vi "Dresden R2R Sputter 03.02.2018 IY24.vi"() -> ()   [LabVIEW 2009] (continued)
                                frame #0 {
                                n25284 = local read "R Set Pressure mtorr"() -> (w30584:dbl)
                                n25285 = local write "Set_pressure_value 2"(w30584) -> ()
                                }
                                frame #1 {
                                }
                                }
                                }
                                frame #1 {
                                n25286 = local read "Semi"() -> (w30585:bool)
                                n25287 = case shown="False" w30585 {
                                frame #0 {
                                n25288 = Wait (ms)(milliseconds to wait=u32 1000) -> ()  [unwired: 1 out]
                                }
                                frame #1 {
                                }
                                }
                                }
                                frame #2 {
                                n25289 = local read "Semi"() -> (w30587:bool)
                                n25290 = case shown="False" w30587 {
                                frame #0 {
                                n25291 = local write "Pc_bv2_auto_set_pressure"(TRUE ("Pc_bv1_auto_set_pressure")) -> ()
                                }
                                frame #1 {
                                }
                                }
                                }
                                frame #3 {
                                n25292 = local read "Semi"() -> (w30589:bool)
                                n25293 = case shown="False" w30589 {
                                frame #0 {
                                n25294 = while {
                                i -> [w30600]
                                stop <- w30592 stop-if-true
                                n25295 = Greater?(x=w30600, y=300) -> (0:w30594:bool)
                                n25296 = local read "Set_pressure_value 2"() -> (w30590:dbl)
                                n25297 = Add(x=1.0, y=w30590) -> (x+y=w30596:dbl)
                                n25298 = Subtract(x=w30590, y=1.0) -> (x-y=w30597:dbl)
                                n25299 = local read "Pressure 2"() -> (w30591:i32)
                                n25300 = In Range and Coerce(upper limit=w30596, x=w30591, lower limit=w30597) -> (In Range?=w30595:bool)  [unwired: 1 out]
                                n25301 = case shown="False" w30595 {
                                tunnel: [FALSE TRUE] -> w30593
                                frame #0 {
                                n25302 = Wait Until Next ms Multiple(millisecond multiple=u32 200) -> ()  [unwired: 1 out]
                                }
                                frame #1 {
                                }
                                }
                                n25303 = Or(x=w30593, y=w30594) -> (x .or. y?=w30592:bool)
                                }
                                }
                                frame #1 {
                                }
                                }
                                }
                                frame #4 {
                                n25304 = local read "Semi"() -> (w30605:bool)
                                n25305 = case shown="False" w30605 {
                                frame #0 {
                                n25306 = local read "Set_pressure_value 2"() -> (w30606:dbl)
                                n25307 = Add(x=1.0, y=w30606) -> (x+y=w30609:dbl)
                                n25308 = Subtract(x=w30606, y=1.0) -> (x-y=w30610:dbl)
                                n25309 = local read "Pressure 2"() -> (w30607:i32)
                                n25310 = In Range and Coerce(upper limit=w30609, x=w30607, lower limit=w30610) -> (In Range?=w30608:bool)  [unwired: 1 out]
                                n25311 = case shown="False" w30608 {
                                frame #0 {
                                n25312 = local read "R Set Pressure mtorr"() -> (w30613:dbl)
                                n25313 = local write "Set_pressure_value 2"(w30613) -> ()
                                }
                                frame #1 {
                                }
                                }
                                }
                                frame #1 {
                                }
                                }
                                }
                                frame #5 {
                                n25314 = local read "Semi"() -> (w30614:bool)
                                n25315 = case shown="False" w30614 {
                                frame #0 {
                                n25316 = local read "Set_pressure_value 2"() -> (w30615:dbl)
                                n25317 = Add(x=1.0, y=w30615) -> (x+y=w30618:dbl)
                                n25318 = Subtract(x=w30615, y=1.0) -> (x-y=w30619:dbl)
                                n25319 = local read "Pressure 2"() -> (w30616:i32)
                                n25320 = In Range and Coerce(upper limit=w30618, x=w30616, lower limit=w30619) -> (In Range?=w30617:bool)  [unwired: 1 out]
                                n25321 = case shown="False" w30617 {
                                frame #0 {
                                n25322 = local write "Pc_bv2_auto_set_pressure"(TRUE ("Pc_bv1_auto_set_pressure")) -> ()
                                }
                                frame #1 {
                                }
                                }
                                }
                                frame #1 {
                                }
                                }
                                }
                                frame #6 {
                                n25323 = local read "Semi"() -> (w30623:bool)
                                n25324 = case shown="False" w30623 {
                                frame #0 {
                                n25325 = while {
                                i -> [w30634]
                                stop <- w30625 stop-if-true
                                n25326 = Greater?(x=w30634, y=300) -> (0:w30627:bool)
                                n25327 = local read "Set_pressure_value 2"() -> (w30629:dbl)
                                n25328 = Add(x=1.0, y=w30629) -> (x+y=w30630:dbl)
                                n25329 = Subtract(x=w30629, y=1.0) -> (x-y=w30631:dbl)
                                n25330 = local read "Pressure 2"() -> (w30624:i32)
                                n25331 = In Range and Coerce(upper limit=w30630, x=w30624, lower limit=w30631) -> (In Range?=w30628:bool)  [unwired: 1 out]
                                n25332 = case shown="False" w30628 {
                                tunnel: [FALSE TRUE] -> w30626
                                frame #0 {
                                n25333 = Wait Until Next ms Multiple(millisecond multiple=u32 200) -> ()  [unwired: 1 out]
                                }
                                frame #1 {
                                }
                                }
                                n25334 = Or(x=w30626, y=w30627) -> (x .or. y?=w30625:bool)
                                }
                                }
                                frame #1 {
                                }
                                }
                                }
                                frame #7 {
                                n25335 = local read "Semi"() -> (w30639:bool)
                                n25336 = case shown="False" w30639 {
                                frame #0 {
                                n25337 = local read "Set_pressure_value 2"() -> (w30642:dbl)
                                n25338 = Add(x=1.0, y=w30642) -> (x+y=w30643:dbl)
                                n25339 = Subtract(x=w30642, y=1.0) -> (x-y=w30644:dbl)
                                n25340 = local read "Pressure 2"() -> (w30640:i32)
                                n25341 = In Range and Coerce(upper limit=w30643, x=w30640, lower limit=w30644) -> (In Range?=w30641:bool)  [unwired: 1 out]
                                n25342 = case shown="False" w30641 {
                                frame #0 {
                                n25343 = local write "Semi"(TRUE ("Semi")) -> ()
                                n25344 = local write "Error Message"("Coating Pressure could not be adjusted !" ("Error Message")) -> ()
                                }
                                frame #1 {
                                }
                                }
                                }
                                frame #1 {
                                }
                                }
                                }
                                }
                                }
                                frame #1 {
                                }
                                }
                                }
                                frame #1 {
                                n25345 = local read "Semi"() -> (w30649:bool)
                                n25346 = case shown="False" w30649 {
                                frame #0 {
                                n25347 = local write "SDC1 9"(TRUE ("SDC1 9")) -> ()
                                n25348 = Wait (ms)(milliseconds to wait=u32 1000) -> ()  [unwired: 1 out]
                                }
                                frame #1 {
                                }
                                }
                                }
                                }
                                }
                                }
                                }
                                frame #15 {
                                # "DC -Ignite Plasma"
                                n25349 = stacked-sequence {
                                frame #0 {
                                n25350 = local read "Semi"() -> (w30652:bool)
                                n25351 = case shown="False" w30652 {
                                frame #0 {
                                n25352 = stacked-sequence {
                                frame #0 {
                                n25353 = local read "Semi"() -> (w30653:bool)
                                n25354 = case shown="False" w30653 {
                                frame #0 {
                                n25355 = while {
                                i -> [w30659]
                                stop <- w30654 stop-if-true
                                n25356 = Greater?(x=w30659, y=50) -> (0:w30658:bool)
                                n25357 = case shown="True" w30658 {
                                frame #0 {
                                }
                                frame #1 {
                                n25358 = local write "Semi"(TRUE ("Semi")) -> ()
                                n25359 = local write "Error Message"("Sputtering Process cancelled.\nPlease check \nDC switch connections." ("Error Message")) -> ()
                                }
                                }
                                n25360 = local read "Cnt_Dcps_sw2_di"() -> (w30657:bool)
                                n25361 = case shown="True" w30657 {
                                tunnel: [TRUE ("Cnt_Dcps_sw1_do") FALSE ("Cnt_Dcps_sw1_do")] -> w30656
                                frame #0 {
                                }
                                frame #1 {
                                n25362 = local write "Cnt_Dcps_sw2_do"(FALSE ("Cnt_Dcps_sw1_do")) -> ()
                                n25363 = Wait Until Next ms Multiple(millisecond multiple=u32 200) -> ()  [unwired: 1 out]
                                }
                                }
                                n25364 = local read "Semi"() -> (w30655:bool)
                                n25365 = Or(x=w30656, y=w30655) -> (x .or. y?=w30654:bool)
                                }
                                }
                                frame #1 {
                                }
                                }
                                }
                                frame #1 {
                                n25366 = local read "Semi"() -> (w30667:bool)
                                n25367 = case shown="False" w30667 {
                                frame #0 {
                                n25368 = while {
                                i -> [w30673]
                                stop <- w30668 stop-if-true
                                n25369 = Greater?(x=w30673, y=50) -> (0:w30672:bool)
                                n25370 = case shown="True" w30672 {
                                frame #0 {
                                }
                                frame #1 {
                                n25371 = local write "Semi"(TRUE ("Semi")) -> ()
                                n25372 = local write "Error Message"("Sputtering Process cancelled.\nPlease check \nDC switch connections." ("Error Message")) -> ()
                                }
                                }
                                n25373 = local read "Cnt_Dcps_sw1_di"() -> (w30671:bool)
                                n25374 = case shown="False" w30671 {
                                tunnel: [FALSE ("Cnt_Dcps_sw1_do") TRUE ("Cnt_Dcps_sw1_do")] -> w30670
                                frame #0 {
                                n25375 = local write "Cnt_Dcps_sw1_do"(TRUE ("Cnt_Dcps_sw1_do")) -> ()
                                n25376 = Wait Until Next ms Multiple(millisecond multiple=u32 200) -> ()  [unwired: 1 out]
                                }
                                frame #1 {
                                }
                                }
                                n25377 = local read "Semi"() -> (w30669:bool)
                                n25378 = Or(x=w30670, y=w30669) -> (x .or. y?=w30668:bool)
                                }
                                }
                                frame #1 {
                                }
                                }
                                }
                                frame #2 {
                                n25379 = local read "Semi"() -> (w30681:bool)
                                n25380 = case shown="False" w30681 {
                                frame #0 {
                                n25381 = local write "Dc_host_auto"(TRUE ("Dc_host_auto")) -> ()
                                }
                                frame #1 {
                                }
                                }
                                }
                                frame #3 {
                                n25382 = local read "Semi"() -> (w30683:bool)
                                n25383 = case shown="False" w30683 {
                                frame #0 {
                                n25384 = local read "R Single DC Step1 Coating Power"() -> (w30684:dbl)
                                n25385 = local write "Set DC Power       :"(w30684) -> ()
                                }
                                frame #1 {
                                }
                                }
                                }
                                frame #4 {
                                n25386 = local read "Semi"() -> (w30685:bool)
                                n25387 = case shown="False" w30685 {
                                frame #0 {
                                n25388 = Wait (ms)(milliseconds to wait=u32 1000) -> ()  [unwired: 1 out]
                                }
                                frame #1 {
                                }
                                }
                                }
                                frame #5 {
                                n25389 = local read "Semi"() -> (w30687:bool)
                                n25390 = case shown="False" w30687 {
                                frame #0 {
                                n25391 = local write "Dc_auto_set"(TRUE ("Dc_auto_set")) -> ()
                                }
                                frame #1 {
                                }
                                }
                                }
                                frame #6 {
                                n25392 = Wait (ms)(milliseconds to wait=u32 1000) -> ()  [unwired: 1 out]
                                }
                                frame #7 {
                                n25393 = local read "Semi"() -> (w30690:bool)
                                n25394 = case shown="False" w30690 {
                                frame #0 {
                                n25395 = local read "Web_selection_tab"() -> (w30691:T5)
                                n25396 = case shown="\"Other                                                                                    \"" w30691 {
                                frame #0 {
                                }
                                frame #1 {
                                n25397 = local write "Dc_auto_on"(TRUE ("Dc_auto_on")) -> ()
                                }
                                }
                                }
                                frame #1 {
                                }
                                }
                                }
                                frame #8 {
                                n25398 = local read "Web_selection_tab"() -> (w30693:T5)
                                n25399 = case shown="\"Other                                                                                    \"" w30693 {
                                frame #0 {
                                }
                                frame #1 {
                                n25400 = local read "Semi"() -> (w30694:bool)
                                n25401 = case shown="False" w30694 {
                                frame #0 {
                                n25402 = while {
                                i -> [w30704]
                                stop <- w30695 stop-if-true
                                n25403 = Greater Or Equal?(x=w30704, y=240) -> (x >= y?=w30703:bool)
                                n25404 = case shown="True" w30703 {
                                frame #0 {
                                }
                                frame #1 {
                                n25405 = local write "Semi"(TRUE ("Semi")) -> ()
                                }
                                }
                                n25406 = local read "Set DC Power       :"() -> (w30700:dbl)
                                n25407 = local read "Actual DC Power"() -> (w30699:dbl)
                                n25408 = Subtract(x=w30700, y=w30699) -> (x-y=w30702:dbl)
                                n25409 = Less?(x=w30702, y=10.0) -> (x < y?=w30697:bool)
                                n25410 = local read "Semi"() -> (w30696:bool)
                                n25411 = Or(x=w30697, y=w30696) -> (x .or. y?=w30695:bool)
                                n25412 = Wait Until Next ms Multiple(millisecond multiple=u32 500) -> ()  [unwired: 1 out]
                                }
                                }
                                frame #1 {
                                }
                                }
                                }
                                }
                                }
                                frame #9 {
                                n25413 = local read "Semi"() -> (w30707:bool)
                                n25414 = case shown="False" w30707 {
                                frame #0 {
                                n25415 = Wait (ms)(milliseconds to wait=u32 1000) -> ()  [unwired: 1 out]
                                }
                                frame #1 {
                                }
                                }
                                }
                                }
                                }
                                frame #1 {
                                }
                                }
                                }
                                frame #1 {
                                n25416 = local read "Semi"() -> (w30709:bool)
                                n25417 = case shown="False" w30709 {
                                frame #0 {
                                n25418 = Wait (ms)(milliseconds to wait=u32 1000) -> ()  [unwired: 1 out]
                                n25419 = local write "SDC1 13"(TRUE ("SDC1 13")) -> ()
                                }
                                frame #1 {
                                }
                                }
                                }
                                }
                                }
                                frame #16 {
                                n25420 = local read "Web_selection_tab"() -> (w30712:T5)
                                n25421 = case shown="\"Web                                                                                    \", Default" w30712 {
                                frame #0 {
                                n25422 = stacked-sequence {
                                frame #0 {
                                n25423 = local read "R Web speed(cm/min)"() -> (w30716:dbl)
                                n25424 = local read "R Minimum diameter"() -> (w30713:dbl)
                                n25425 = local read "R Maximum diameter"() -> (w30714:dbl)
                                n25426 = local read "R Web thicness"() -> (w30715:dbl)
                                n25427 = local write "Initial Min Diameter"(w30713) -> ()
                                n25428 = local write "Web Thickness"(w30715) -> ()
                                n25429 = local write "Max Diameter"(w30714) -> ()
                                n25430 = local write "Web Speed"(w30716) -> ()
                                n25431 = Wait (ms)(milliseconds to wait=u32 100) -> ()  [unwired: 1 out]
                                }
                                frame #1 {
                                n25432 = local read "R Single DC Step1 Coating Power Active"() -> (w30731:bool)
                                n25433 = local read "R Single DC Step2 Coating Power Active"() -> (w30730:bool)
                                n25434 = local read "R Single DC Step3 Coating Power Active"() -> (w30729:bool)
                                n25435 = local read "R Single DC Step4 Coating Power Active"() -> (w30728:bool)
                                n25436 = local read "R Single DC Step5 Coating Power Active"() -> (w30727:bool)
                                n25437 = Boolean To (0,1)(Boolean=w30731) -> (0, 1=w30726:i16)
                                n25438 = Boolean To (0,1)(Boolean=w30730) -> (0, 1=w30725:i16)
                                n25439 = Boolean To (0,1)(Boolean=w30729) -> (0, 1=w30724:i16)
                                n25440 = Boolean To (0,1)(Boolean=w30728) -> (0, 1=w30723:i16)
                                n25441 = Boolean To (0,1)(Boolean=w30727) -> (0, 1=w30722:i16)
                                n25442 = Compound Arithmetic op=ADD(w30726, w30725, w30724, w30723, w30722) -> (w30720:i16)
                                n25443 = local read "R Single DC Interval length"() -> (w30721:dbl)
                                n25444 = Wait (ms)(milliseconds to wait=u32 200) -> ()  [unwired: 1 out]
                                n25445 = Multiply(x=w30721, y=w30720) -> (x*y=w30719:dbl)
                                n25446 = local write "Total length"(w30719) -> ()
                                }
                                frame #2 {
                                n25447 = local write "Calculate 2"(TRUE ("Calculate_auto")) -> ()
                                }
                                frame #3 {
                                n25448 = local write "Roll_side_select"(enum32{"Left to Right", "Right to Left"}."Left to Right" ("Roll_side_select")) -> ()
                                }
                                frame #4 {
                                n25449 = Wait (ms)(milliseconds to wait=u32 100) -> ()  [unwired: 1 out]
                                n25450 = local write "Parameters_auto_set"(TRUE ("Parameters_auto_set")) -> ()
                                }
                                frame #5 {
                                n25451 = while {
                                i -> [w30740]
                                stop <- w30736 stop-if-true
                                n25452 = Wait Until Next ms Multiple(millisecond multiple=u32 300) -> ()  [unwired: 1 out]
                                n25453 = Greater?(x=w30740, y=100) -> (0:w30737:bool)
                                n25454 = local read "Parameters_auto_set"() -> (w30741:bool)
                                n25455 = case shown="False" w30741 {
                                tunnel: [TRUE FALSE] -> w30738
                                frame #0 {
                                }
                                frame #1 {
                                }
                                }
                                n25456 = Or(x=w30738, y=w30737) -> (x .or. y?=w30736:bool)
                                }
                                }
                                frame #6 {
                                n25457 = local read "R Tension Value"() -> (w30745:dbl)
                                n25458 = Wait (ms)(milliseconds to wait=u32 200) -> ()  [unwired: 1 out]
                                n25459 = local write "TC1_set_value"(w30745) -> ()
                                }
                                frame #7 {
                                n25460 = local write "TC1_auto_set"(TRUE ("TC1_auto_set")) -> ()
                                }
                                frame #8 {
                                w30749 = u16 1 items=["1", "2", "3", "4"] ("Target Chamber Sensor")
                                n25461 = local write "Target Chamber Sensor"(w30749) -> ()
                                n25462 = Wait (ms)(milliseconds to wait=u32 200) -> ()  [unwired: 1 out]
                                }
                                frame #9 {
                                n25463 = local read "Total length"() -> (w30750:dbl)
                                n25464 = local write "Region"(w30750) -> ()
                                }
                                frame #10 {
                                n25465 = local read "Semi"() -> (w30751:bool)
                                n25466 = case shown="False" w30751 {
                                frame #0 {
                                n25467 = stacked-sequence {
                                frame #0 {
                                # "Gas Flow"
                                n25468 = stacked-sequence {
                                frame #0 {
                                n25469 = local read "Semi"() -> (w30752:bool)
                                n25470 = case shown="False" w30752 {
                                frame #0 {
                                n25471 = stacked-sequence {
                                frame #0 {
                                n25472 = local read "Semi"() -> (w30753:bool)
                                n25473 = case shown="False" w30753 {
                                frame #0 {
                                n25474 = local read "R Argon Flow sccm"() -> (w30754:dbl)
                                n25475 = local write "Ar_sccm1_2"(w30754) -> ()
                                }
                                frame #1 {
                                }
                                }
                                }
                                frame #1 {
                                n25476 = local read "Semi"() -> (w30755:bool)
                                n25477 = case shown="False" w30755 {
                                frame #0 {
                                n25478 = local write "Mfc_Ar _1_2_set"(TRUE ("Mfc_Ar _1_2_set")) -> ()
                                }
                                frame #1 {
                                }
                                }
                                }
                                frame #2 {
                                n25479 = local read "Semi"() -> (w30757:bool)
                                n25480 = case shown="False" w30757 {
                                frame #0 {
                                n25481 = while {
                                i -> [w30760]
                                stop <- w30762 stop-if-true
                                n25482 = Greater?(x=w30760, y=50) -> (0:w30759:bool)
                                n25483 = local read "Semi"() -> (w30758:bool)
                                n25484 = Or(x=w30758, y=w30759) -> (x .or. y?=w30762:bool)
                                }
                                }
                                frame #1 {
                                }
                                }
                                }
                                frame #3 {
                                n25485 = local read "Semi"() -> (w30763:bool)
                                n25486 = case shown="False" w30763 {
                                frame #0 {
                                n25487 = local read "Ar_sccm_act 6"() -> (w30764:dbl)
                                n25488 = Greater?(x=w30764, y=1) -> (0:w30765:bool)
                                n25489 = case shown="False" w30765 {
                                frame #0 {
                                n25490 = local read "R Argon Flow sccm"() -> (w30767:dbl)
                                n25491 = local write "Ar_sccm1_2"(w30767) -> ()
                                }
                                frame #1 {
                                }
                                }
                                }
                                frame #1 {
                                }
                                }
                                }
                                frame #4 {
                                n25492 = local read "Semi"() -> (w30768:bool)
                                n25493 = case shown="False" w30768 {
                                frame #0 {
                                n25494 = local read "Ar_sccm_act 6"() -> (w30770:dbl)
                                n25495 = Greater?(x=w30770, y=1) -> (0:w30769:bool)
                                n25496 = case shown="False" w30769 {
                                frame #0 {
                                n25497 = while {
                                i -> [w30773]
                                stop <- w30777 stop-if-true
                                n25498 = Greater?(x=w30773, y=50) -> (0:w30772:bool)
                                n25499 = local read "Semi"() -> (w30776:bool)
                                n25500 = case shown="False" w30776 {
                                tunnel: [FALSE TRUE] -> w30775
                                frame #0 {
                                n25501 = Wait Until Next ms Multiple(millisecond multiple=u32 200) -> ()  [unwired: 1 out]
                                }
                                frame #1 {
                                }
                                }
                                n25502 = Or(x=w30775, y=w30772) -> (x .or. y?=w30777:bool)
                                }
                                }
                                frame #1 {
                                }
                                }
                                }
                                frame #1 {
                                }
                                }
                                }
                                frame #5 {
                                n25503 = local read "Semi"() -> (w30781:bool)
                                n25504 = case shown="False" w30781 {
                                frame #0 {
                                n25505 = local read "Ar_sccm_act 5"() -> (w30783:dbl)
                                n25506 = Greater?(x=w30783, y=1) -> (0:w30782:bool)
                                n25507 = case shown="False" w30782 {
                                frame #0 {
                                n25508 = local write "Semi"(TRUE ("Semi")) -> ()
                                n25509 = local write "Error Message"("Coating process cancelled.\nPlease check connections." ("Error Message")) -> ()
                                }
                                frame #1 {
                                }
                                }
                                }
                                frame #1 {
                                }
                                }
                                }
                                }
                                }
                                frame #1 {
                                }
                                }
                                }
                                frame #1 {
                                n25510 = local read "Semi"() -> (w30787:bool)
                                n25511 = case shown="False" w30787 {
                                frame #0 {
                                n25512 = local write "SDC1 11"(TRUE ("SDC1 11")) -> ()
                                n25513 = Wait (ms)(milliseconds to wait=u32 1000) -> ()  [unwired: 1 out]
                                }
                                frame #1 {
                                }
                                }
                                }
                                }
                                }
                                frame #1 {
                                # "Set Pressure for ignite plasma"
                                n25514 = stacked-sequence {
                                frame #0 {
                                n25515 = local read "Semi"() -> (w30790:bool)
                                n25516 = case shown="False" w30790 {
                                frame #0 {
                                n25517 = stacked-sequence {
                                frame #0 {
                                n25518 = local read "Semi"() -> (w30791:bool)
                                n25519 = case shown="False" w30791 {
                                frame #0 {
                                n25520 = local write "Set_pressure_value 2"(10.0 ("Set_pressure_value 2")) -> ()
                                }
                                frame #1 {
                                }
                                }
                                }
                                frame #1 {
                                n25521 = local read "Semi"() -> (w30793:bool)
                                n25522 = case shown="False" w30793 {
                                frame #0 {
                                n25523 = Wait (ms)(milliseconds to wait=u32 1000) -> ()  [unwired: 1 out]
                                }
                                frame #1 {
                                }
                                }
                                }
                                frame #2 {
                                n25524 = local read "Semi"() -> (w30795:bool)
                                n25525 = case shown="False" w30795 {
                                frame #0 {
                                n25526 = local write "Pc_bv2_auto_set_pressure"(TRUE ("Pc_bv1_auto_set_pressure")) -> ()
                                }
                                frame #1 {
                                }
                                }
                                }
                                frame #3 {
                                n25527 = local read "Semi"() -> (w30797:bool)
                                n25528 = case shown="False" w30797 {
                                frame #0 {
                                n25529 = while {
                                i -> [w30808]
                                stop <- w30800 stop-if-true
                                w30798 = 10.0 ("Set_pressure_value 2")
                                n25530 = Greater?(x=w30808, y=300) -> (0:w30802:bool)
                                n25531 = Add(x=1.0, y=w30798) -> (x+y=w30804:dbl)
                                n25532 = Subtract(x=w30798, y=1.0) -> (x-y=w30805:dbl)
                                n25533 = local read "Pressure 2"() -> (w30799:i32)
                                n25534 = In Range and Coerce(upper limit=w30804, x=w30799, lower limit=w30805) -> (In Range?=w30803:bool)  [unwired: 1 out]
                                n25535 = case shown="False" w30803 {
                                tunnel: [FALSE TRUE] -> w30801
                                frame #0 {
                                n25536 = Wait Until Next ms Multiple(millisecond multiple=u32 200) -> ()  [unwired: 1 out]
                                }
                                frame #1 {
                                }
                                }
                                n25537 = Or(x=w30801, y=w30802) -> (x .or. y?=w30800:bool)
                                }
                                }
                                frame #1 {
                                }
                                }
                                }
                                frame #4 {
                                n25538 = local read "Semi"() -> (w30813:bool)
                                n25539 = case shown="False" w30813 {
                                frame #0 {
                                w30814 = 10.0 ("Set_pressure_value 2")
                                n25540 = Add(x=1.0, y=w30814) -> (x+y=w30817:dbl)
                                n25541 = Subtract(x=w30814, y=1.0) -> (x-y=w30818:dbl)
                                n25542 = local read "Pressure 2"() -> (w30815:i32)
                                n25543 = In Range and Coerce(upper limit=w30817, x=w30815, lower limit=w30818) -> (In Range?=w30816:bool)  [unwired: 1 out]
                                n25544 = case shown="False" w30816 {
                                frame #0 {
                                n25545 = local read "R Set Pressure mtorr"() -> (w30821:dbl)
                                n25546 = local write "Set_pressure_value 2"(w30821) -> ()
                                }
                                frame #1 {
                                }
                                }
                                }
                                frame #1 {
                                }
                                }
                                }
                                frame #5 {
                                n25547 = local read "Semi"() -> (w30822:bool)
                                n25548 = case shown="False" w30822 {
                                frame #0 {
                                w30823 = 10.0 ("Set_pressure_value 2")
                                n25549 = Add(x=1.0, y=w30823) -> (x+y=w30826:dbl)
                                n25550 = Subtract(x=w30823, y=1.0) -> (x-y=w30827:dbl)
                                n25551 = local read "Pressure 2"() -> (w30824:i32)
                                n25552 = In Range and Coerce(upper limit=w30826, x=w30824, lower limit=w30827) -> (In Range?=w30825:bool)  [unwired: 1 out]
                                n25553 = case shown="False" w30825 {
                                frame #0 {
                                n25554 = local write "Pc_bv2_auto_set_pressure"(TRUE ("Pc_bv1_auto_set_pressure")) -> ()
                                }
                                frame #1 {
                                }
                                }
                                }
                                frame #1 {
                                }
                                }
                                }
                                frame #6 {
                                n25555 = local read "Semi"() -> (w30831:bool)
                                n25556 = case shown="False" w30831 {
                                frame #0 {
                                n25557 = while {
                                i -> [w30842]
                                stop <- w30834 stop-if-true
                                w30832 = 10.0 ("Set_pressure_value 2")
                                n25558 = Greater?(x=w30842, y=300) -> (0:w30836:bool)
                                n25559 = Add(x=1.0, y=w30832) -> (x+y=w30838:dbl)
                                n25560 = Subtract(x=w30832, y=1.0) -> (x-y=w30839:dbl)
                                n25561 = local read "Pressure 2"() -> (w30833:i32)
                                n25562 = In Range and Coerce(upper limit=w30838, x=w30833, lower limit=w30839) -> (In Range?=w30837:bool)  [unwired: 1 out]
                                n25563 = case shown="False" w30837 {
                                tunnel: [FALSE TRUE] -> w30835
                                frame #0 {
                                n25564 = Wait Until Next ms Multiple(millisecond multiple=u32 200) -> ()  [unwired: 1 out]
                                }
                                frame #1 {
                                }
                                }
                                n25565 = Or(x=w30835, y=w30836) -> (x .or. y?=w30834:bool)
                                }
                                }
                                frame #1 {
                                }
                                }
                                }
                                frame #7 {
                                n25566 = local read "Semi"() -> (w30847:bool)
                                n25567 = case shown="False" w30847 {
                                frame #0 {
                                n25568 = local read "Set_pressure_value 2"() -> (w30850:dbl)
                                n25569 = Add(x=1.0, y=w30850) -> (x+y=w30851:dbl)
                                n25570 = Subtract(x=w30850, y=1.0) -> (x-y=w30852:dbl)
                                n25571 = local read "Pressure 2"() -> (w30848:i32)
                                n25572 = In Range and Coerce(upper limit=w30851, x=w30848, lower limit=w30852) -> (In Range?=w30849:bool)  [unwired: 1 out]
                                n25573 = case shown="False" w30849 {
                                frame #0 {
                                n25574 = local write "Semi"(TRUE ("Semi")) -> ()
                                n25575 = local write "Error Message"("Coating Pressure could not be adjusted !" ("Error Message")) -> ()
                                }
                                frame #1 {
                                }
                                }
                                }
                                frame #1 {
                                }
                                }
                                }
                                }
                                }
                                frame #1 {
                                }
                                }
                                }
                                frame #1 {
                                n25576 = local read "Semi"() -> (w30857:bool)
                                n25577 = case shown="False" w30857 {
                                frame #0 {
                                n25578 = local write "SDC1 9"(TRUE ("SDC1 9")) -> ()
                                n25579 = Wait (ms)(milliseconds to wait=u32 1000) -> ()  [unwired: 1 out]
                                }
                                frame #1 {
                                }
                                }
                                }
                                }
                                }
                                frame #2 {
                                # "Plasma ignite and check"
                                n25580 = stacked-sequence {
                                frame #0 {
                                n25581 = local read "Semi"() -> (w30860:bool)
                                n25582 = case shown="False" w30860 {
                                frame #0 {
                                n25583 = local write "Dc_auto_on"(TRUE ("Dc_auto_on")) -> ()